vi "tempVoltageAndImpeadance1.vi"() -> ()   [LabVIEW 2018]
panel:
  out "Tab Control":T1(tab)
  in  "File Location Directory":string="C:\\Research"
  in  "VNA":bool
  in  "Scope and Opsens":bool
  in  "ModulePath":path=path "C:/Research/Sena's CodeBase and Documents/tempsScopeAndVNALabview.py"
  in  "scopeReadFunction":string="scopeRead"
  in  "opsensReadFunction":string="opsensRead"
  in  "vnaFunctionName":string="vnaRead"
  in  "dataFileWriteFunction":string="writeDataFiles"
  in  "writeImpeadanceFiles":string="writeImpeadanceData"
  out "error out":errorcluster
  out "Program Executed":bool
  out "Oscilloscope Channel 1 Output Graph":cluster{dbl[], dbl[]}[](graph)
  in  "shortRecordLength":i32=10000
  in  "scopeNumCollects":i32=3
  in  "longRecordLength 2":i32=100000
  in  "numChan":i32=2
  out "scopeErrorOut":errorcluster
  out "Opsens Channel 1":cluster{"Array 2":dbl[], "Array 3":dbl[]}[](graph)
  out "Oscilloscope Channel 2 Output Graph":cluster{dbl[], dbl[]}[](graph)
  out "opsensErrorOut":errorcluster
  out "writeImpeadanceFilesError":errorcluster
  out "Vector Network Analyzer Graph":cluster{dbl[], dbl[]}(graph)
  in  "vnaNumOfRecordings":dbl=5001.0
  in  "vnaStartFreq":dbl=100000.0
  in  "vnaEndFreq":dbl=30000000.0
  out "vnaErrorOut":errorcluster
  out "Program Executed":bool
  # "Note:\nThe Vector Network Analyzer will still run if both conditions\nare both true or both false."
  # "Opsens PicoM Controls"
  # "Oscilloscope Controls"
  # "Vector Network Analyzer Controls"
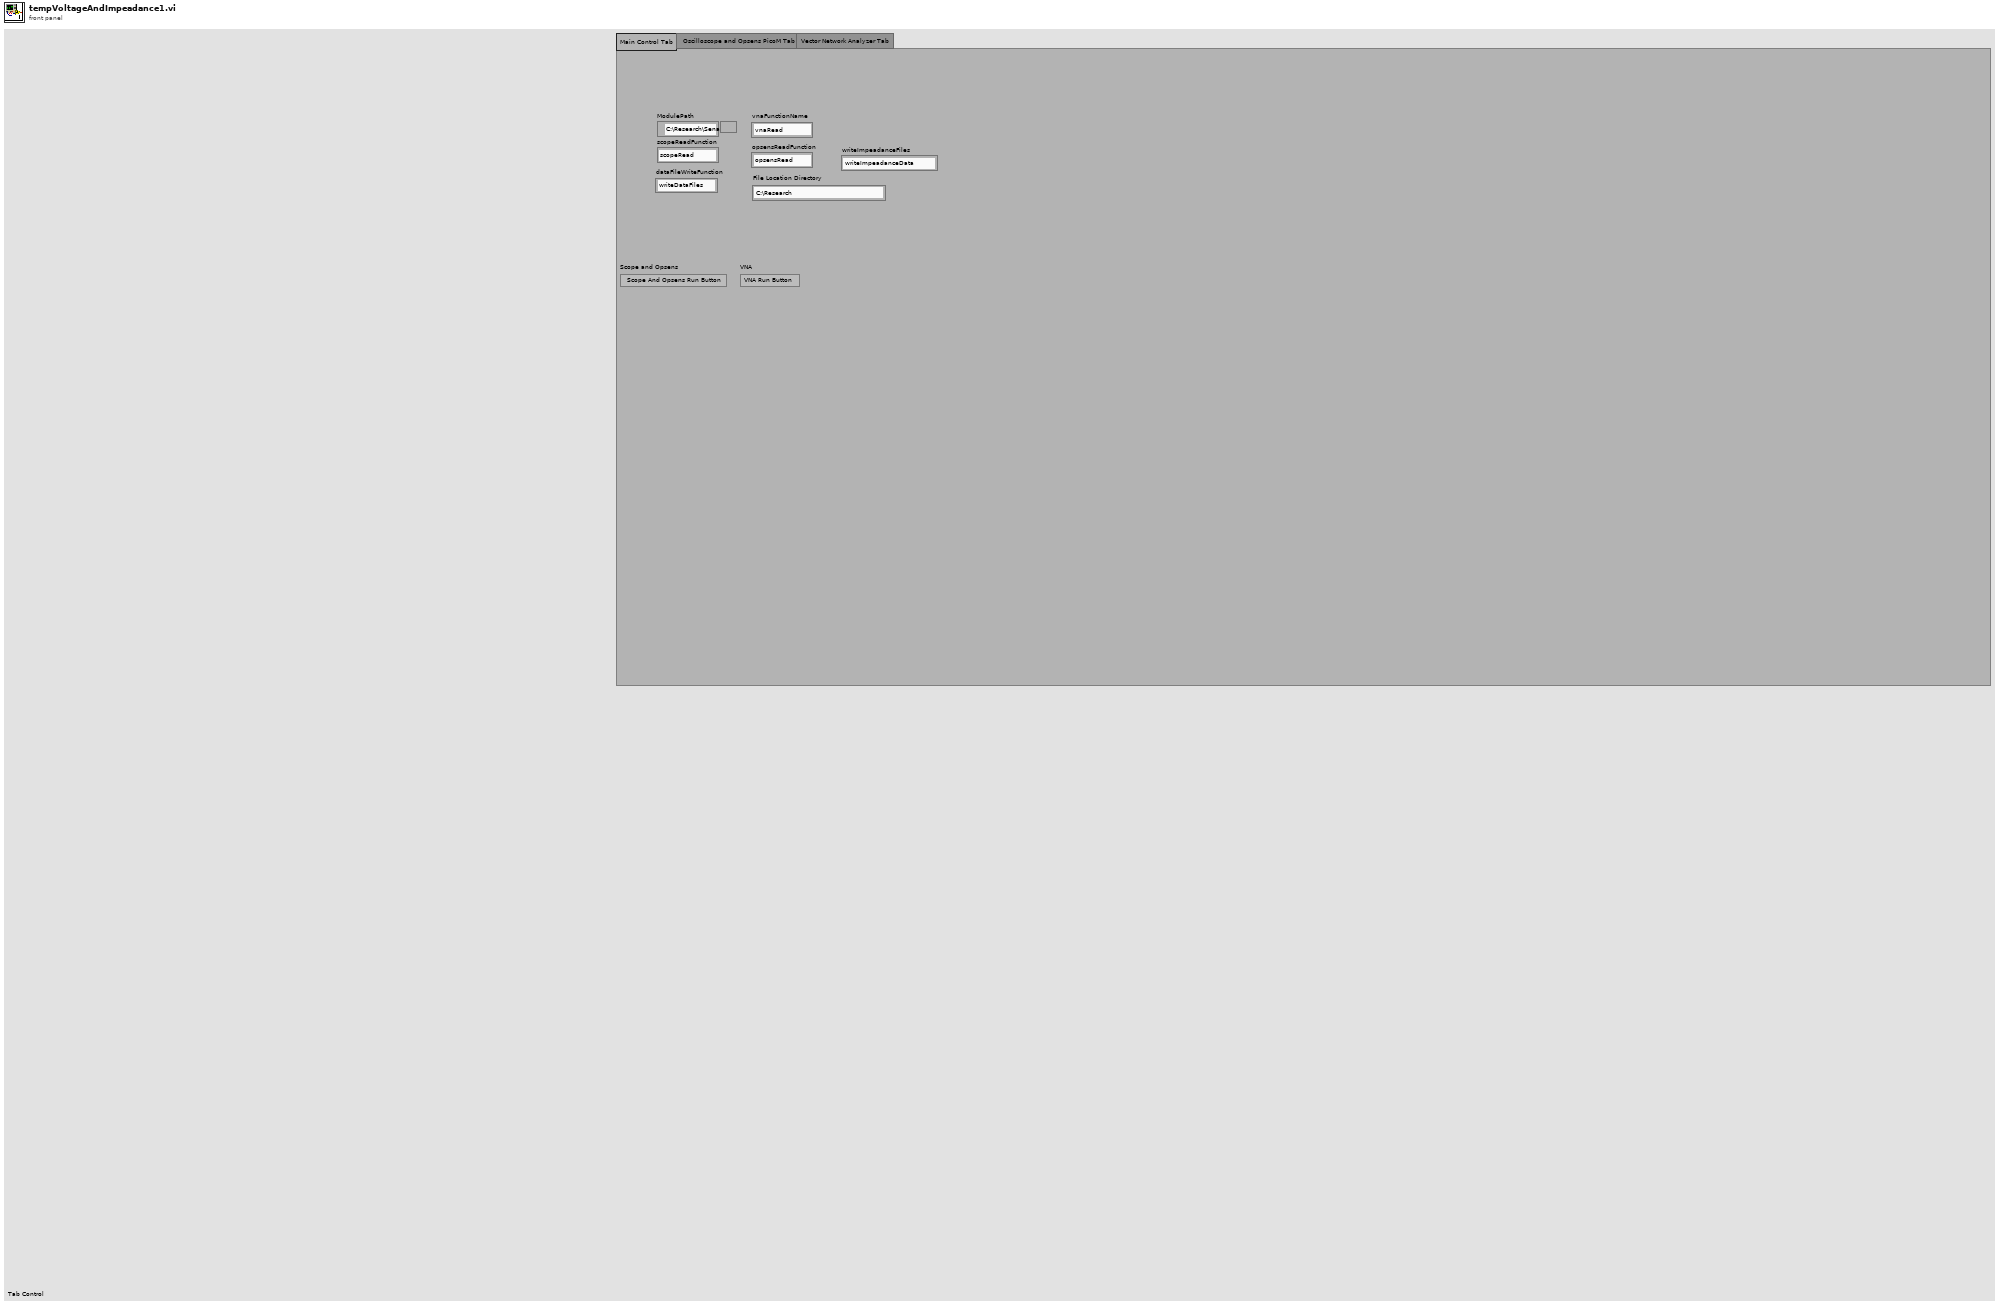
[diagram p1: front panel]
types:
  T1 = enum32{"Main Control Tab", " Oscilloscope and Opsens PicoM Tab", "Vector Network Analyzer Tab"}
  T2 = enum16{"Main Control Tab", "Oscilloscope and Opsens PicoM Tab", "Vector Network Analyzer Tab"}
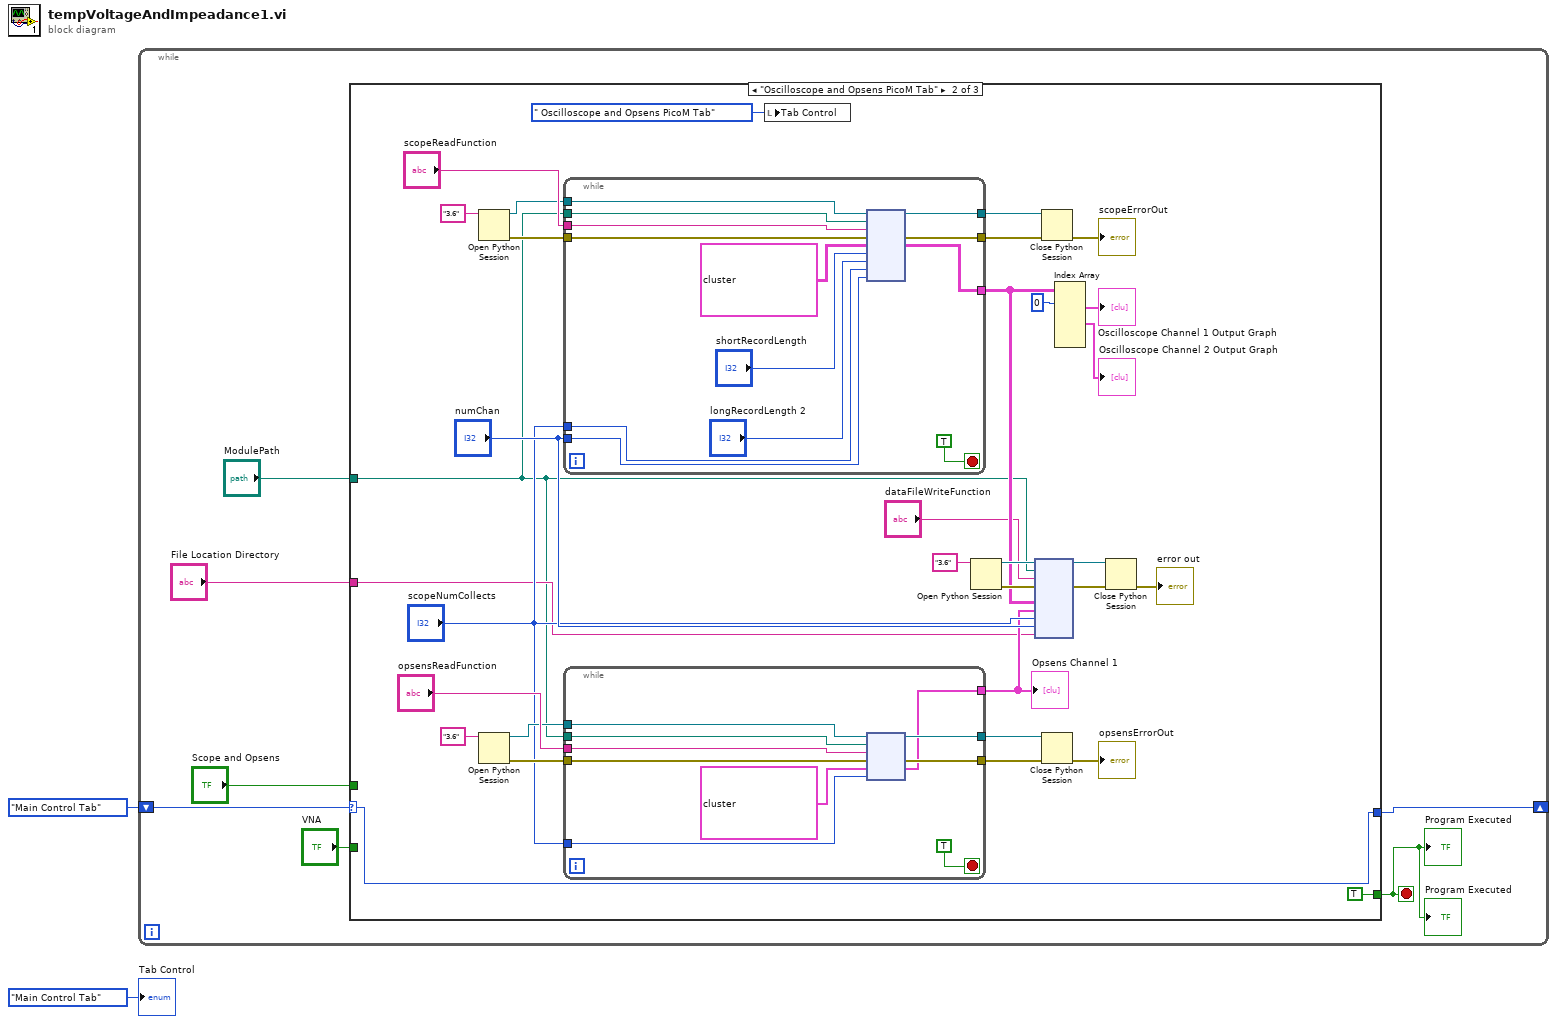
[diagram p0: block diagram]
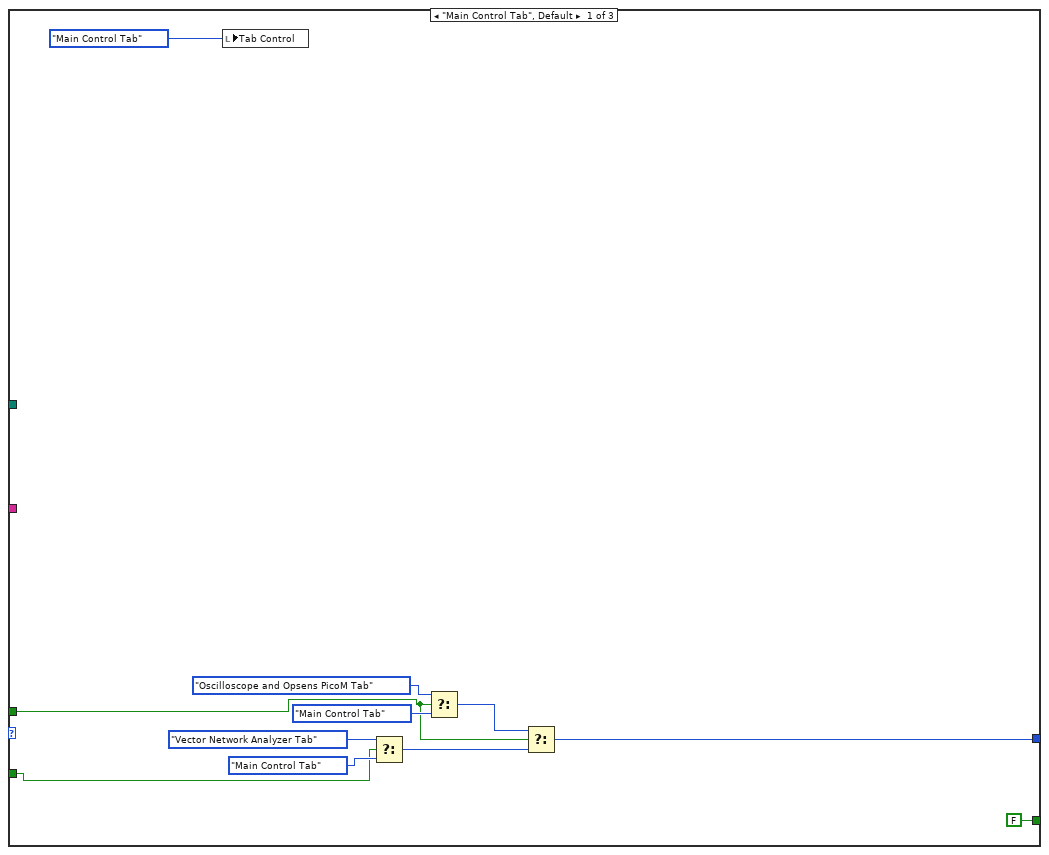
[diagram p2: hidden frame]
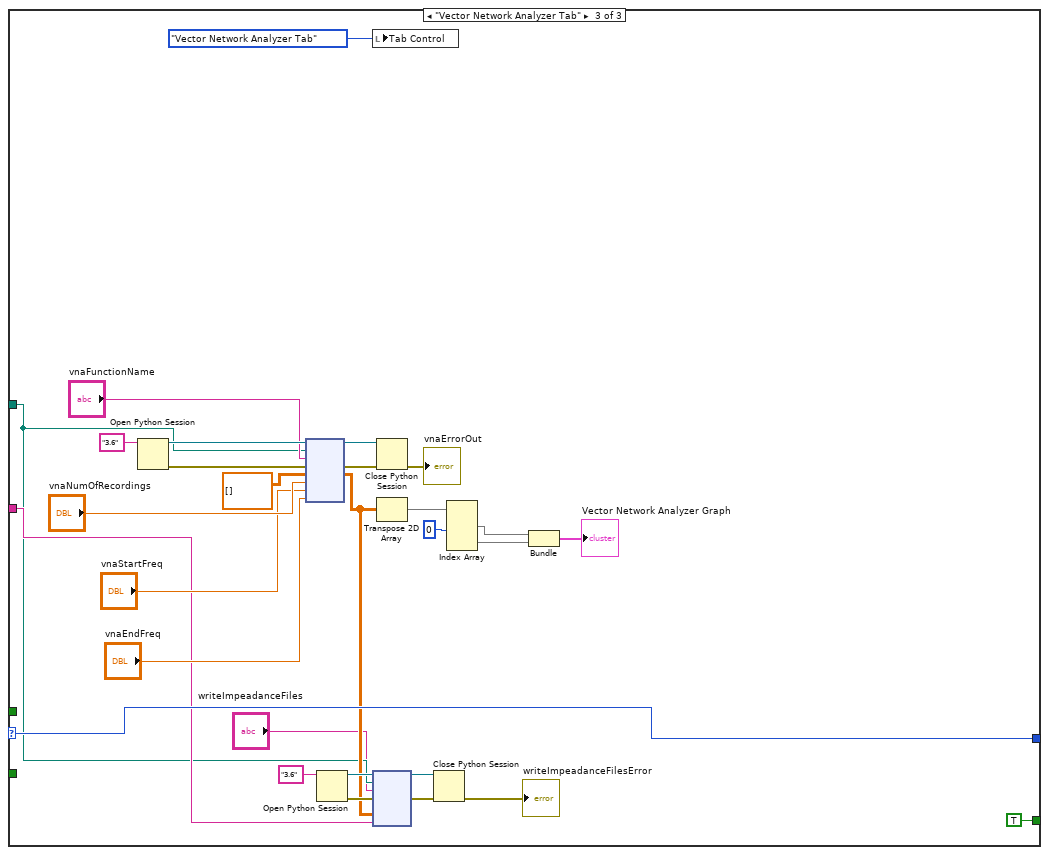
[diagram p3: hidden frame]
diagram:
  n1 = while {
    shift-right: [w6] -> _
    shift-left: T2."Main Control Tab" -> [w9]
    stop <- w5 stop-if-true
    n2 = case shown="\"Oscilloscope and Opsens PicoM Tab\"" w9 {
      selector: w9 -> [_ w52 w104]
      tunnel: "Scope and Opsens" -> [w14 _ _]
      tunnel: "VNA" -> [w13 _ _]
      tunnel: [w12 w52 w104] -> w6
      tunnel: [FALSE TRUE TRUE] -> w5
      tunnel: "File Location Directory" -> [_ w22 w81]
      tunnel: "ModulePath" -> [_ w21 w80]
      frame "Main Control Tab", Default {
        n3 = local write "Tab Control"(T1."Main Control Tab" ("Tab Control")) -> ()
        n4 = Select(t=T2."Vector Network Analyzer Tab", s=w13, f=T2."Main Control Tab") -> (s? t:f=w15:T2)
        n5 = Select(t=T2."Oscilloscope and Opsens PicoM Tab", s=w14, f=T2."Main Control Tab") -> (s? t:f=w16:T2)
        n6 = Select(t=w16, s=w14, f=w15) -> (s? t:f=w12:T2)
      }
      frame "Oscilloscope and Opsens PicoM Tab" {
        n7 = Open Python Session(python version="3.6" ("Python version")) -> (session out=w40:refnum<k35>, error out=w43:errorcluster)  [unwired: 2 in]
        n8 = Open Python Session(python version="3.6") -> (session out=w44:refnum<k35>, error out=w47:errorcluster)  [unwired: 2 in]
        n9 = while {
          tunnel: w40 -> [w73]
          tunnel: [w72] -> w41
          tunnel: [w71] -> w42
          tunnel: w43 -> [w70]
          tunnel: w21 -> [w69]
          tunnel: "scopeReadFunction" -> [w68]
          tunnel: [w67] -> w27
          tunnel: "scopeNumCollects" -> [w65]
          tunnel: "numChan" -> [w64]
          stop <- TRUE stop-if-true
          n10 = node(w73, w69, w68, w70, cluster{"Array 2":dbl[], "Array 3":dbl[]}[][] [[{"Array 2"=array[100000 elements], "Array 3"=array[100000 elements]}, {"Array 2"=array[100000 elements], "Array 3"=array[100000 elements]}, {"Array 2"=array[100000 elements], "Array 3"=array[100000 elements]}]] ("Array 2"), "shortRecordLength", "longRecordLength 2", w65, w64) -> (w72:refnum<k35>, w71:errorcluster, w67:cluster{"Array 2":dbl[], "Array 3":dbl[]}[][])  [unwired: 4 in, 2 out]
        }
        n11 = while {
          tunnel: w44 -> [w62]
          tunnel: [w61] -> w45
          tunnel: [w60] -> w46
          tunnel: w47 -> [w59]
          tunnel: w21 -> [w58]
          tunnel: "opsensReadFunction" -> [w57]
          tunnel: "scopeNumCollects" -> [w56]
          tunnel: [w54] -> w26
          stop <- TRUE stop-if-true
          n12 = node(w62, w58, w57, w59, cluster{"Array 2":dbl[], "Array 3":dbl[]}[] [{"Array 2"=array[100000 elements], "Array 3"=array[100000 elements]}, {"Array 2"=array[100000 elements], "Array 3"=array[100000 elements]}, {"Array 2"=array[100000 elements], "Array 3"=array[100000 elements]}] ("Array 2"), w56) -> (w61:refnum<k35>, w60:errorcluster, w54:cluster{"Array 2":dbl[], "Array 3":dbl[]}[])  [unwired: 1 in, 2 out]
        }
        "Opsens Channel 1" <- w26
        n13 = local write "Tab Control"(T1." Oscilloscope and Opsens PicoM Tab" ("Tab Control")) -> ()
        n14 = Open Python Session(python version="3.6" ("Python version")) -> (session out=w33:refnum<k35>, error out=w32:errorcluster)  [unwired: 2 in]
        n15 = node(w33, w21, "dataFileWriteFunction", w32, w27, w26, "scopeNumCollects", "numChan", w22) -> (w31:refnum<k35>, w30:errorcluster)  [unwired: 7 in, 2 out]
        n16 = Close Python Session(session in=w41, error in=w42) -> (11:→"scopeErrorOut":errorcluster)
        n17 = Close Python Session(session in=w45, error in=w46) -> (11:→"opsensErrorOut":errorcluster)
        n18 = Index Array(array=w27, index (row) #1=0 ("index (page)")) -> (element #1=→"Oscilloscope Channel 1 Output Graph":cluster{"Array 2":dbl[], "Array 3":dbl[]}[], element #2=→"Oscilloscope Channel 2 Output Graph":cluster{"Array 2":dbl[], "Array 3":dbl[]}[])  [unwired: 5 in, 1 out]
        n19 = Close Python Session(session in=w31, error in=w30) -> (11:→"error out":errorcluster)
      }
      frame "Vector Network Analyzer Tab" {
        n20 = Open Python Session(python version="3.6" ("Python version")) -> (session out=w100:refnum<k35>, error out=w101:errorcluster)  [unwired: 2 in]
        n21 = node(w100, w80, "vnaFunctionName", w101, dbl[][] [], "vnaNumOfRecordings", "vnaStartFreq", "vnaEndFreq") -> (w102:refnum<k35>, w103:errorcluster, w82:dbl[][])  [unwired: 3 in, 2 out]
        n22 = Open Python Session(python version="3.6" ("Python version")) -> (session out=w86:refnum<k35>, error out=w84:errorcluster)  [unwired: 2 in]
        n23 = local write "Tab Control"(T1."Vector Network Analyzer Tab" ("Tab Control")) -> ()
        n24 = node(w86, w80, "writeImpeadanceFiles", w84, w82, w81) -> (w85:refnum<k35>, w83:errorcluster)  [unwired: 4 in, 2 out]
        n25 = Close Python Session(session in=w102, error in=w103) -> (11:→"vnaErrorOut":errorcluster)
        n26 = Transpose 2D Array(2D array=w82) -> (transposed array=w93:dbl[][])
        n27 = Close Python Session(session in=w85, error in=w83) -> (11:→"writeImpeadanceFilesError":errorcluster)
        n28 = Index Array(array=w93, index (col) #1=0 ("length")) -> (element #1=w92:dbl[], element #2=w91:dbl[])  [unwired: 3 in]
        n29 = Bundle(w92, w91) -> (→"Vector Network Analyzer Graph":cluster{dbl[], dbl[]})  [unwired: 1 in]
      }
    }
    "Program Executed" <- w5
    "Program Executed" <- w5
  }
  "Tab Control" <- T1."Main Control Tab" ("Tab Control")
